vi "IMAQdx_AbsImage_Flea3_v4.5.vi"() -> ()   [LabVIEW 2013] (continued)
+combWidthF/2))\tODTpowHLat(DipPowHLat)\t1\tVimaging\t0\t0\t0\t1\t1\t1\tbMOTdelta(MOTdetuning)\tbMOTpow(0.5)\tProbePow\t0\tXshim\tYshim\tZshimVar\tODTpowZ(DipPowZ)\tVimaging\t0\t0\tHimaging\t0\t0\t0\t0\t0\t0\t0\t0\t0\t0\t0\t0\t0\t0\trMOTdelta(-(rMOTstirDetI +stirWidthF/2))\t0\tODTpowXY(DipPowCr)\tvarWaveP2\t0\t0\trMOTpow3\tODTpowX(DipPowX)\tfreq\tHeatingAmp\t0\tSine\tDetuning\tsingleFreqDet\tDoppCoolDet-DoppCoolSweep\tdopCoolT*1000\tDetuning\tsingleFreqStirDet\tsingleFreqStirDet + 20\tSFcoolT*1000\tBlueBN\tBlueLaserProbeBN\tPixisPos(TOF)\tCycle Wait for Move\tEOMmodFreq\tEOMmodAmp\r\ntransmit img\t\tRamp\t1\t.6\t0\t0\t0\t0\t0\t0\t1\t0\t0\t1\t0\t0\t0\t0\t0\t0\t0\t0\t0\t0\t0\t0\t0\t0\t0\t0\t1\t0\t0\t0\t1\t1\t0\tplus_zman\tminus_zman\tcompensation\trMOTcurrF\trMOTpow3\tcombAmplitude(combWidthF)\trMOTdelta(-(rMOTbroadDetuningF +combWidthF/2))\tODTpowHLat(DipPowHLat)\t1\tVimaging\t0\t0\t0\t1\t1\t1\tbMOTdelta(MOTdetuning)\tbMOTpow(0.5)\tProbePow\t0\tXshim\tYshim\tZshimVar\tODTpowZ(DipPowZ)\tVimaging\t0\t0\tHimaging\t0\t0\t0\t0\t0\t0\t0\t0\t0\t0\t0\t0\t0\t0\trMOTdelta(-(rMOTstirDetI +stirWidthF/2))\t0\tODTpowXY(DipPowCr)\tvarWaveP2\t0\t0\trMOTpow3\tODTpowX(DipPowX)\tfreq\tHeatingAmp\t0\tSine\tDetuning\tsingleFreqDet\tDoppCoolDet-DoppCoolSweep\tdopCoolT*1000\tDetuning\tsingleFreqStirDet\tsingleFreqStirDet + 20\tSFcoolT*1000\tBlueBN\tBlueLaserProbeBN\tPixisPos(TOF)\tCycle Wait for Move\tEOMmodFreq\tEOMmodAmp\r\narm PIXIS\t\tRamp\t0\t.007\t0\t0\t0\t0\t0\t0\t1\t0\t0\t1\t1\t0\t0\t0\t1\t1\t0\t0\t0\t0\t0\t0\t0\t0\t0\t0\t1\t0\t0\t0\t1\t1\t0\tplus_zman\tminus_zman\tcompensation\trMOTcurrF\trMOTpow1\tcombAmplitude(combWidthF)\trMOTdelta(-(rMOTbroadDetuningF +combWidthF/2))\tODTpowHLat(DipPowHLat)\t1\tVimaging\t0\t0\t0\t1\t1\t1\tbMOTdelta(MOTdetuning)\tbMOTpow(0.5)\tProbePow\t0\tXshim\tYshim\tZshimVar\tODTpowZ(DipPowZ)\tVimaging\t0\t0\tHimaging\t0\t0\t0\t0\t0\t0\t0\t0\t0\t0\t0\t0\t0\t0\trMOTdelta(-(rMOTstirDetI +stirWidthF/2))\t0\tODTpowXY(DipPowCr)\tvarWaveP2\t0\t0\trMOTpow1\tODTpowX(DipPowX)\tfreq\tHeatingAmp\t0\tSine\tDetuning\tsingleFreqDet\tDoppCoolDet-DoppCoolSweep\tdopCoolT*1000\tDetuning\tsingleFreqStirDet\tsingleFreqStirDet + 20\tSFcoolT*1000\tBlueBN\tBlueLaserProbeBN\tPixisPos(TOF)\tCycle Wait for Move\tEOMmodFreq\tEOMmodAmp\r\narm FLEA\t\tRamp\t1\t44e-6\t0\t0\t0\t0\t0\t0\t1\t0\t0\t1\t1\t0\t0\t0\t1\t1\t0\t0\t0\t0\t0\t0\t0\t0\t0\t0\t1\t0\t0\t0\t1\t0\t0\tplus_zman\tminus_zman\tcompensation\trMOTcurrF\trMOTpow1\tcombAmplitude(combWidthF)\trMOTdelta(-(rMOTbroadDetuningF +combWidthF/2))\tODTpowHLat(DipPowHLat)\t1\tVimaging\t0\t0\t0\t1\t1\t0\tbMOTdelta(MOTdetuning)\tbMOTpow(0.5)\tProbePow\t0\tXshim\tYshim\tZshimVar\tODTpowZ(DipPowZ)\tVimaging\t0\t0\tHimaging\t0\t0\t0\t0\t0\t0\t0\t0\t0\t0\t0\t0\t0\t0\trMOTdelta(-(rMOTstirDetI +stirWidthF/2))\t0\tODTpowXY(DipPowCr)\tvarWaveP2\t0\t0\trMOTpow1\tODTpowX(DipPowX)\tfreq\tHeatingAmp\t0\tSine\tDetuning\tsingleFreqDet\tDoppCoolDet-DoppCoolSweep\tdopCoolT*1000\tDetuning\tsingleFreqStirDet\tsingleFreqStirDet + 20\tSFcoolT*1000\tBlueBN\tBlueLaserProbeBN\tPixisPos(TOF)\tCycle Wait for Move\tEOMmodFreq\tEOMmodAmp\r\nprobe img\t\tRamp\t1\t10e-6\t0\t0\t0\t0\t0\t0\t1\t0\t1\t1\t1\t0\t0\t1\t1\t1\t0\t0\t0\t0\t0\t0\t0\t0\t0\t0\t1\t0\t0\t0\t1\t0\t0\tplus_zman\tminus_zman\tcompensation\trMOTcurrF\trMOTpow1\tcombAmplitude(combWidthF)\trMOTdelta(-(rMOTbroadDetuningF +combWidthF/2))\tODTpowHLat(DipPowHLat)\t1\tVimaging\t0\t0\t0\t1\t0\t0\tbMOTdelta(MOTdetuning)\tbMOTpow(0.5)\tProbePow\t0\tXshim\tYshim\tZshimVar\tODTpowZ(DipPowZ)\tVimaging\t0\t0\tHimaging\t0\t0\t0\t0\t0\t0\t0\t0\t0\t0\t0\t0\t0\t0\trMOTdelta(-(rMOTstirDetI +stirWidthF/2))\t0\tODTpowXY(DipPowCr)\tvarWaveP2\t0\t0\trMOTpow1\tODTpowX(DipPowX)\tfreq\tHeatingAmp\t0\tSine\tDetuning\tsingleFreqDet\tDoppCoolDet-DoppCoolSweep\tdopCoolT*1000\tDetuning\tsingleFreqStirDet\tsingleFreqStirDet + 20\tSFcoolT*1000\tBlueBN\tBlueLaserProbeBN\tPixisPos(TOF)\tCycle Wait for Move\tEOMmodFreq\tEOMmodAmp\r\nprobe img\t\tRamp\t0\t2.8e-3\t0\t0\t0\t0\t0\t0\t1\t0\t0\t1\t1\t0\t0\t0\t1\t1\t0\t0\t0\t0\t0\t0\t0\t0\t0\t0\t1\t0\t0\t0\t1\t1\t0\tplus_zman\tminus_zman\tcompensation\trMOTcurrF\trMOTpow1\tcombAmplitude(combWidthF)\trMOTdelta(-(rMOTbroadDetuningF +combWidthF/2))\tODTpowHLat(DipPowHLat)\t1\tVimaging\t0\t0\t0\t1\t1\t1\tbMOTdelta(MOTdetuning)\tbMOTpow(0.5)\tProbePow\t0\tXshim\tYshim\tZshimVar\tODTpowZ(DipPowZ)\tVimaging\t0\t0\tHimaging\t0\t0\t0\t0\t0\t0\t0\t0\t0\t0\t0\t0\t0\t0\trMOTdelta(-(rMOTstirDetI +stirWidthF/2))\t0\tODTpowXY(DipPowCr)\tvarWaveP2\t0\t0\trMOTpow1\tODTpowX(DipPowX)\tfreq\tHeatingAmp\t0\tSine\tDetuning\tsingleFreqDet\tDoppCoolDet-DoppCoolSweep\tdopCoolT*1000\tDetuning\tsingleFreqStirDet\tsingleFreqStirDet + 20\tSFcoolT*1000\tBlueBN\tBlueLaserProbeBN\tPixisPos(TOF)\tCycle Wait for Move\tEOMmodFreq\tEOMmodAmp\r\ntransmit img\t\tRamp\t1\t.585\t0\t0\t0\t0\t0\t0\t1\t0\t0\t1\t1\t0\t0\t0\t1\t1\t0\t0\t0\t0\t0\t0\t0\t0\t0\t0\t1\t0\t0\t0\t1\t1\t0\tplus_zman\tminus_zman\tcompensation\trMOTcurrF\trMOTpow1\tcombAmplitude(combWidthF)\trMOTdelta(-(rMOTbroadDetuningF +combWidthF/2))\tODTpowHLat(DipPowHLat)\t1\tVimaging\t0\t0\t0\t1\t1\t1\tbMOTdelta(MOTdetuning)\tbMOTpow(0.5)\tProbePow\t0\tXshim\tYshim\tZshimVar\tODTpowZ(DipPowZ)\tVimaging\t0\t0\tHimaging\t0\t0\t0\t0\t0\t0\t0\t0\t0\t0\t0\t0\t0\t0\trMOTdelta(-(rMOTstirDetI +stirWidthF/2))\t0\tODTpowXY(DipPowCr)\tvarWaveP2\t0\t0\trMOTpow1\tODTpowX(DipPowX)\tfreq\tHeatingAmp\t0\tSine\tDetuning\tsingleFreqDet\tDoppCoolDet-DoppCoolSweep\tdopCoolT*1000\tDetuning\tsingleFreqStirDet\tsingleFreqStirDet + 20\tSFcoolT*1000\tBlueBN\tBlueLaserProbeBN\tPixisPos(TOF)\tCycle Wait for Move\tEOMmodFreq\tEOMmodAmp\r\ntransmit img\t\tRamp\t1\t.015\t0\t0\t0\t0\t0\t0\t1\t0\t0\t1\t1\t0\t0\t0\t1\t1\t0\t0\t0\t0\t0\t0\t0\t0\t0\t0\t1\t0\t0\t0\t1\t1\t0\tplus_zman\tminus_zman\tcompensation\trMOTcurrF\trMOTpow1\tcombAmplitude(combWidthF)\trMOTdelta(-(rMOTbroadDetuningF +combWidthF/2))\tODTpowHLat(DipPowHLat)\t1\tVimaging\t0\t0\t0\t1\t1\t1\tbMOTdelta(MOTdetuning)\tbMOTpow(0.5)\tProbePow\t0\tXshim\tYshim\tZshimVar\tODTpowZ(DipPowZ)\tVimaging\t0\t0\tHimaging\t0\t0\t0\t0\t0\t0\t0\t0\t0\t0\t0\t0\t0\t0\trMOTdelta(-(rMOTstirDetI +stirWidthF/2))\t0\tODTpowXY(DipPowCr)\tvarWaveP2\t0\t0\trMOTpow1\tODTpowX(DipPowX)\tfreq\tHeatingAmp\t0\tSine\tDetuning\tsingleFreqDet\tDoppCoolDet-DoppCoolSweep\tdopCoolT*1000\tDetuning\tsingleFreqStirDet\tsingleFreqStirDet + 20\tSFcoolT*1000\tBlueBN\tBlueLaserProbeBN\tPixisPos(TOF)\tCycle Wait for Move\tEOMmodFreq\tEOMmodAmp\r\narm PIXIS\t\tRamp\t0\t.007\t0\t0\t0\t0\t0\t0\t1\t0\t0\t1\t1\t0\t0\t0\t1\t1\t0\t0\t0\t0\t0\t0\t0\t0\t0\t0\t1\t0\t0\t0\t1\t0\t0\tplus_zman\tminus_zman\tcompensation\trMOTcurrF\trMOTpow1\tcombAmplitude(combWidthF)\trMOTdelta(-(rMOTbroadDetuningF +combWidthF/2))\tODTpowHLat(DipPowHLat)\t1\tVimaging\t0\t0\t0\t1\t1\t1\tbMOTdelta(MOTdetuning)\tbMOTpow(0.5)\tProbePow\t0\tXshim\tYshim\tZshimVar\tODTpowZ(DipPowZ)\tVimaging\t0\t0\tHimaging\t0\t0\t0\t0\t0\t0\t0\t0\t0\t0\t0\t0\t0\t0\trMOTdelta(-(rMOTstirDetI +stirWidthF/2))\t0\tODTpowXY(DipPowCr)\tvarWaveP2\t0\t0\trMOTpow1\tODTpowX(DipPowX)\tfreq\tHeatingAmp\t0\tSine\tDetuning\tsingleFreqDet\tDoppCoolDet-DoppCoolSweep\tdopCoolT*1000\tDetuning\tsingleFreqStirDet\tsingleFreqStirDet + 20\tSFcoolT*1000\tBlueBN\tBlueLaserProbeBN\tPixisPos(TOF)\tCycle Wait for Move\tEOMmodFreq\tEOMmodAmp\r\narm FLEA\t\tRamp\t1\t44e-6\t0\t0\t0\t0\t0\t0\t1\t0\t0\t1\t1\t0\t0\t0\t1\t1\t0\t0\t0\t0\t0\t0\t0\t0\t0\t0\t1\t0\t0\t0\t1\t0\t0\tplus_zman\tminus_zman\tcompensation\trMOTcurrF\trMOTpow1\tcombAmplitude(combWidthF)\trMOTdelta(-(rMOTbroadDetuningF +combWidthF/2))\tODTpowHLat(DipPowHLat)\t1\tVimaging\t0\t0\t0\t1\t1\t0\tbMOTdelta(MOTdetuning)\tbMOTpow(0.5)\tProbePow\t0\tXshim\tYshim\tZshimVar\tODTpowZ(DipPowZ)\tVimaging\t0\t0\tHimaging\t0\t0\t0\t0\t0\t0\t0\t0\t0\t0\t0\t0\t0\t0\trMOTdelta(-(rMOTstirDetI +stirWidthF/2))\t0\tODTpowXY(DipPowCr)\tvarWaveP2\t0\t0\trMOTpow1\tODTpowX(DipPowX)\tfreq\tHeatingAmp\t0\tSine\tDetuning\tsingleFreqDet\tDoppCoolDet-DoppCoolSweep\tdopCoolT*1000\tDetuning\tsingleFreqStirDet\tsingleFreqStirDet + 20\tSFcoolT*1000\tBlueBN\tBlueLaserProbeBN\tPixisPos(TOF)\tCycle Wait for Move\tEOMmodFreq\tEOMmodAmp\r\nbg img\t\tRamp\t1\t10e-6\t0\t0\t0\t0\t0\t0\t1\t0\t0\t1\t1\t0\t0\t0\t1\t1\t0\t0\t0\t0\t0\t0\t0\t0\t0\t0\t1\t0\t0\t0\t1\t0\t0\tplus_zman\tminus_zman\tcompensation\trMOTcurrF\trMOTpow1\tcombAmplitude(combWidthF)\trMOTdelta(-(rMOTbroadDetuningF +combWidthF/2))\tODTpowHLat(DipPowHLat)\t1\tVimaging\t0\t0\t0\t1\t0\t0\tbMOTdelta(MOTdetuning)\tbMOTpow(0.5)\tProbePow\t0\tXshim\tYshim\tZshimVar\tODTpowZ(DipPowZ)\tVimaging\t0\t0\tHimaging\t0\t0\t0\t0\t0\t0\t0\t0\t0\t0\t0\t0\t0\t0\trMOTdelta(-(rMOTstirDetI +stirWidthF/2))\t0\tODTpowXY(DipPowCr)\tvarWaveP2\t0\t0\trMOTpow1\tODTpowX(DipPowX)\tfreq\tHeatingAmp\t0\tSine\tDetuning\tsingleFreqDet\tDoppCoolDet-DoppCoolSweep\tdopCoolT*1000\tDetuning\tsingleFreqStirDet\tsingleFreqStirDet + 20\tSFcoolT*1000\tBlueBN\tBlueLaserProbeBN\tPixisPos(TOF)\tCycle Wait for Move\tEOMmodFreq\tEOMmodAmp\r\nbg img\t\tRamp\t0\t1e-4\t0\t0\t0\t0\t0\t0\t1\t0\t0\t1\t1\t0\t0\t0\t1\t1\t0\t0\t0\t0\t0\t0\t0\t0\t0\t0\t1\t0\t0\t0\t1\t1\t0\tplus_zman\tminus_zman\tcompensation\trMOTcurrF\trMOTpow1\tcombAmplitude(combWidthF)\trMOTdelta(-(rMOTbroadDetuningF +combWidthF/2))\tODTpowHLat(DipPowHLat)\t1\tVimaging\t0\t0\t0\t1\t1\t1\tbMOTdelta(MOTdetuning)\tbMOTpow(0.5)\tProbePow\t0\tXshim\tYshim\tZshimVar\tODTpowZ(DipPowZ)\tVimaging\t0\t0\tHimaging\t0\t0\t0\t0\t0\t0\t0\t0\t0\t0\t0\t0\t0\t0\trMOTdelta(-(rMOTstirDetI +stirWidthF/2))\t0\tODTpowXY(DipPowCr)\tvarWaveP2\t0\t0\trMOTpow1\tODTpowX(DipPowX)\tfreq\tHeatingAmp\t0\tSine\tDetuning\tsingleFreqDet\tDoppCoolDet-DoppCoolSweep\tdopCoolT*1000\tDetuning\tsingleFreqStirDet\tsingleFreqStirDet + 20\tSFcoolT*1000\tBlueBN\tBlueLaserProbeBN\tPixisPos(TOF)\tCycle Wait for Move\tEOMmodFreq\tEOMmodAmp\r\ntransmit img\t\tRamp\t1\t.6\t0\t0\t0\t0\t0\t0\t1\t0\t0\t1\t1\t0\t0\t0\t1\t1\t0\t0\t0\t0\t0\t0\t0\t0\t0\t0\t1\t0\t0\t0\t1\t1\t0\tplus_zman\tminus_zman\tcompensation\trMOTcurrF\trMOTpow1\tcombAmplitude(combWidthF)\trMOTdelta(-(rMOTbroadDetuningF +combWidthF/2))\tODTpowHLat(DipPowHLat)\t1\tVimaging\t0\t0\t0\t1\t1\t1\tbMOTdelta(MOTdetuning)\tbMOTpow(0.5)\tProbePow\t0\tXshim\tYshim\tZshimVar\tODTpowZ(DipPowZ)\tVimaging\t0\t0\tHimaging\t0\t0\t0\t0\t0\t0\t0\t0\t0\t0\t0\t0\t0\t0\trMOTdelta(-(rMOTstirDetI +stirWidthF/2))\t0\tODTpowXY(DipPowCr)\tvarWaveP2\t0\t0\trMOTpow1\tODTpowX(DipPowX)\tfreq\tHeatingAmp\t0\tSine\tDetuning\tsingleFreqDet\tDoppCoolDet-DoppCoolSweep\tdopCoolT*1000\tDetuning\tsingleFreqStirDet\tsingleFreqStirDet + 20\tSFcoolT*1000\tBlueBN\tBlueLaserProbeBN\tPixisPos(TOF)\tCycle Wait for Move\tEOMmodFreq\tEOMmodAmp\r\nalignment\t\tRamp\t1\t.1\t1\t1\t1\t1\t1\t1\t1\t0\t1\t0\t1\t0\t1\t1\t1\t1\t0\t0\t0\t0\t0\t0\t0\t0\t1m\t0\t1\t0\t1\t0\t0\t1\t1\tplus_zman\tminus_zman\tcompensation\tMOTcurrent\trMOTpow1\tcombAmplitude(combWidthI)\trMOTdelta(-(rMOTbroadDetuningI +combWidthI/2))\tODTpowHLat(DipPowHLat)\t1\t0\t1\t1\t0\t1\t1\t1\tbMOTdelta(MOTdetuning)\tbMOTpow(MOTPow)\tProbePow\t0\tXshim\tYshim\tZshim\tODTpowZ(DipPowZ2)\t0\t1\t0\t0\t1\t1\t0\t0\t0\t0\t0\t0\t0\t0\t0\t0\t0\t0\trMOTdelta(-(rMOTstirDetI +stirWidthI/2))\t0\tODTpowXY(DipPowCr)\tvarWaveP2\t0\t0\trMOTpow3\tODTpowX(DipPowX)\tfreq\tHeatingAmp\t0\tSine\tRamp\tsingleFreqDet\tsingleFreqDetF\tSFcoolT*1000\tRamp\tsingleFreqStirDet\tsingleFreqStirDetF\tSFcoolT*1000\tBlueBN\tBlueLaserBeatnote\tPixisPos(TOF)\tCycle Wait for Move\tEOMmodFreq\tEOMmodAmp\r\n\r\n\r\n"
  in  "Flea Wave Name":string="Test_Img"
  in  "Save files to archive?":bool
  out "Timeout":bool=TRUE
  out "Trigger Overrun":bool=TRUE
  in  "Source of File Data":refnum<k21>="\\\\192.168.137.181\\VariableLibrary\\Instruction String"
  in  "Timeout (ms)":u32=20000
  in  "Gain":dbl
  in  "Shutter speed":dbl=0.03
  in  "PIXIS Magnification":dbl=5.48
  in  "PIXIS Image direction":enum16{"XY", "XZ"}(ring)
  in  "PIXIS Imaging technique":enum16{"Absorption", "Fluorescence", "RawImage"}(ring)
  in  "SPE File Path":path=path "C:/Users/Lab/Documents/LightField/LabviewTemp.spe"
  in  "Send PIXIS data to Igor?":bool
  in  "PIXIS File Parameters":T1={"Data Root"=path "I:/Data", "Index"=4, "Instrument"="PIXIS"} {"Index" format="%04d"}
  in  "Source of Wavemeter Data":refnum<k21>="\\\\WS7PC\\VariableLibrary\\Frequency"
  in  "Accept wavelength from remote system":bool=TRUE
  in  "Flea Raw image to view":u16(ring) items=["Clear", "Absorbtion", "Probe", "Background"]
  in  "Update Graphics":bool=TRUE
  out "Flea Raw Image":u16[][](graph)
  out "Flea Processed Image":sgl[][](graph)
  out "PIXIS Processed Image":sgl[][](graph)
  out "PIXIS Raw Image":u16[][](graph)
  in  "PIXIS Raw image to view":u16(ring)=1 items=["Clear", "Absorbtion", "Probe", "Background"]
  out "Camera Error":errorcluster={"status"=FALSE, "code"=-1074360293, "source"="IMAQdx Get Image2.vi"}
  out "DDE Error":errorcluster={"status"=TRUE, "code"=14012, "source"="DDE Execute: DMLERR_NOTPROCESSED"}
  out "Status Array":T4(array[cluster])=[{"AcquisitionInProgress"=FALSE, "BufferCount"=0, "LastBufferNumber"=4294967292, "LostBufferCount"=0}, {"AcquisitionInProgress"=TRUE, "BufferCount"=0, "LastBufferNumber"=4294967292, "LostBufferCount"=0}, {"AcquisitionInProgress"=TRUE, "BufferCount"=1, "LastBufferNumber"=0, "LostBufferCount"=0}, {"AcquisitionInProgress"=TRUE, "BufferCount"=2, "LastBufferNumber"=1, "LostBufferCount"=0}, {"AcquisitionInProgress"=TRUE, "BufferCount"=3, "LastBufferNumber"=2, "LostBufferCount"=0}, {"AcquisitionInProgress"=TRUE, "BufferCount"=4, "LastBufferNumber"=3, "LostBufferCount"=0}]
  in  "SPE Load Error In":errorcluster
  out "DataBlock Info":T5={"frame count"=4, "frame size"=524288, "frame stride"=524288, "N ROI"=1, "ROI widths"=[512], "ROI heights"=[512], "ROI sizes"=[524288], "ROI strides"=[524288]}
  out "DS Error":errorcluster
  out "XML Parse Errors":string
  out "Data Array Size":i32=1
  out "SPE Load Error Out":errorcluster
  out "Flea Path":path=path "I:/Data/Flea3_20S4Mtemp.ibw"
  out "PIXIS Path":path=path "C:/Experiment/Data/PIXIStemp.ibw"
  out "PIXIS Images":u16[][][](array[numeric])
  out "Flea Images":u16[][][](array[numeric])
  out "Buffer Number":u32=4294967294
  out "Flea Frames":i32
  out "Flea Loop":i32=1
  # "Image Acquisition v4.5"
  # "Experimental Parameters"
  # "These are only get set on 1st run.\nUse a Gain of 0, Shutter Speed not used"
  # "In both techniques 3 images\nare aquired, but in Fluorescense\nthe 3rd is discarded"
  # "Sr: .663  is XZ a\n     .898 is XZ b\n      5.48 is XY"
  # "Obsolete: (now done with network variables)\nWhen paramaters are accepted from a remote system a DataSockets server\nmust be running on this machine (in start menu in National Instruments folder)"
  # "Camera configuration"
  # "File configuration"
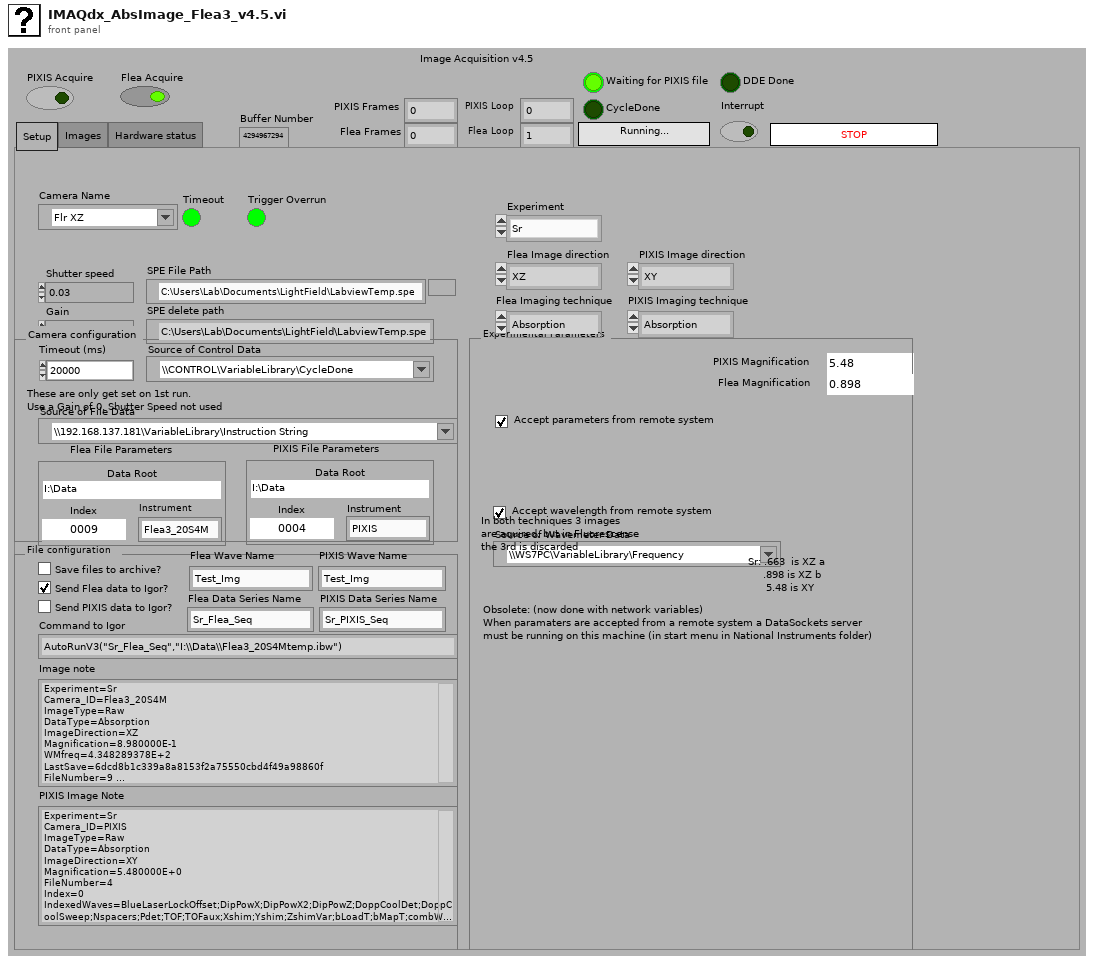
[diagram p1: front panel]
types:
  T1 = typedef "FileName_Cluster.ctl" = cluster{"Data Root":path, "Index":u32, "Instrument":string}
  T2 = typedef "IMAQdx.ctl" = refnum<k21>
  T3 = enum16{"Rubidium I", "Rubidium II", "RbLi", "RbYb", "Sr"}
  T4 = cluster{"AcquisitionInProgress":bool, "BufferCount":u32, "LastBufferNumber":u32, "LostBufferCount":u32}[]
  T5 = cluster{"frame count":i64, "frame size":i64, "frame stride":i64, "N ROI":i64, "ROI widths":i64[], "ROI heights":i64[], "ROI sizes":i64[], "ROI strides":i64[]}
  T6 = typedef "NI_Vision_Acquisition_Software.lvlib/IMAQdx Acquisition Mode.ctl" = enum32{"One Shot", "Continuous"}
  T7 = typedef "Image Type" = u32
  T8 = typedef "IMAQ Image.ctl" = refnum<image>
  T9 = cluster{"AcquisitionInProgress":bool, "BufferCount":u32, "LastBufferNumber":u32, "LostBufferCount":u32}
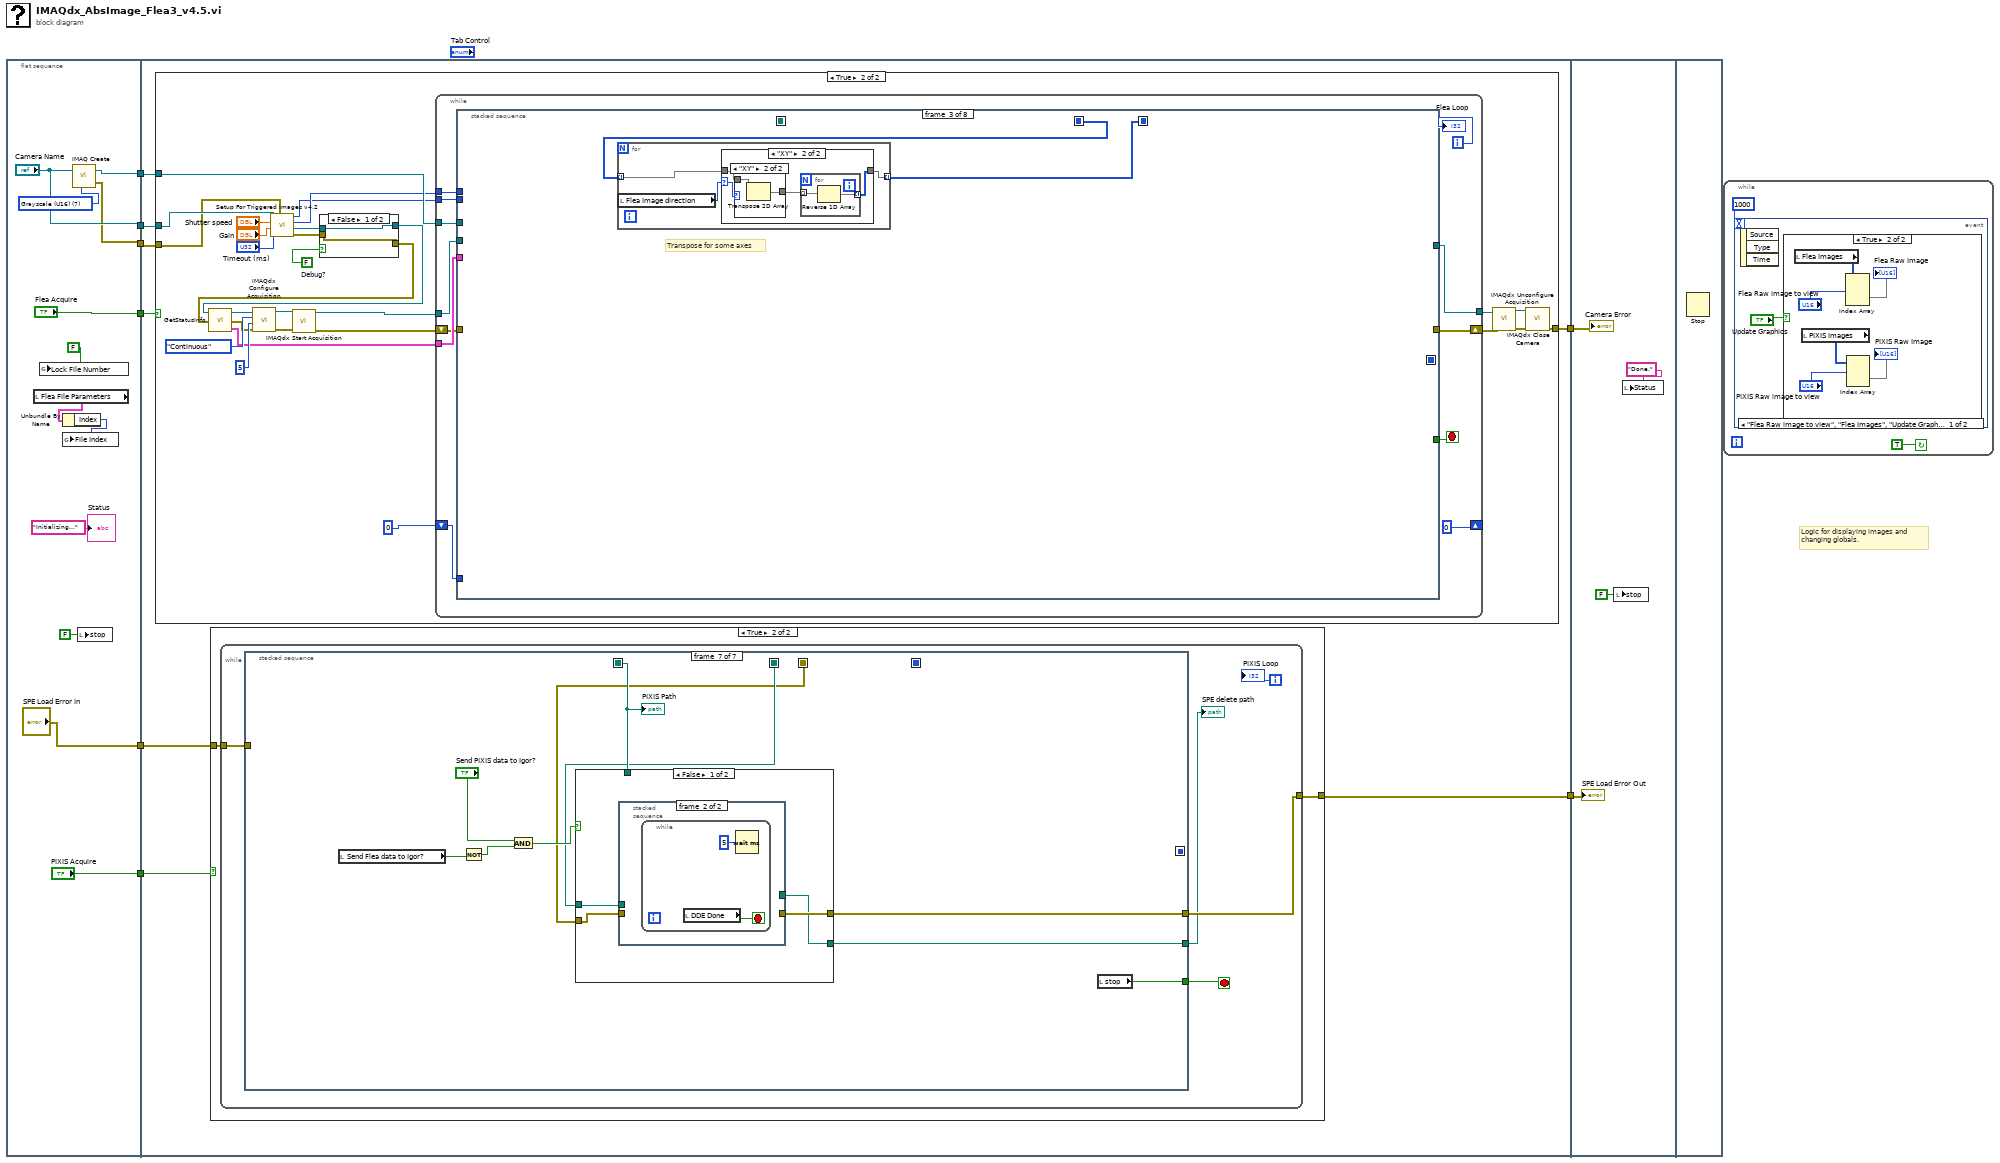
[diagram p0: block diagram]
diagram:
  # "Logic for displaying images and\nchanging globals."
  n1 = flat-sequence {
    tunnel: [w16] -> w8
    tunnel: ["Camera Name"] -> w7
    tunnel: [w14] -> w6
    tunnel: ["SPE Load Error In"] -> w5
    tunnel: ["PIXIS Acquire"] -> w3
    tunnel: ["Flea Acquire"] -> w1
    tunnel: w7 -> [w28]
    tunnel: w8 -> [w26]
    tunnel: w6 -> [w27]
    tunnel: w5 -> [w25]
    tunnel: [w24] -> w4
    tunnel: w3 -> [w23]
    tunnel: [w22] -> w2
    tunnel: w1 -> [w21]
    tunnel: w4 -> [w463]
    tunnel: w2 -> [w462]
    frame #0 {
      w13 = T7 7 items=["Grayscale (U8)", "Grayscale (I16)", "Grayscale (SGL)", "Complex (CSG)", "RGB (U32)", "HSL (U32)", "RGB (U64)", "Grayscale (U16)"] ("Image Type")
      n2 = local read "Flea File Parameters"() -> (w17:T1)
      n3 = global write "FileInfo_Global.vi" "Lock File Number"(FALSE) -> ()
      n4 = Unbundle By Name(w17) -> ("Index"=w18:u32)
      n5 = global write "FileInfo_Global.vi" "File Index"(w18) -> ()
      n6 = call "IMAQ Create"("Image Name"="Camera Name", "Image Type"=w13) -> ("New Image"=w16:T8, "error out"=w14:errorcluster)  [unwired: 2 in, 1 out]
      n7 = local write "stop"(FALSE ("stop")) -> ()
      "Status" <- "Initializing..."
    }
    frame #1 {
      n8 = case shown="True" w21 {
        tunnel: w28 -> [_ w43]
        tunnel: w27 -> [w29 w42]
        tunnel: w26 -> [_ w40]
        tunnel: [w29 w32] -> w22
        frame False {
        }
        frame True {
          w50 = FALSE  # Debug?
          n9 = call "Setup For Triggered Images v4.2.vi"("error in"=w42, "Timeout (ms)"="Timeout (ms)", "Gain"="Gain", "Shutter speed"="Shutter speed", "Camera Name"=w43) -> ("Error out"=w51:errorcluster, "Session Out"=w52:T2, "Height"=w39:u32, "Width"=w38:u32)
          n10 = case shown="False" w50 {
            tunnel: [w58 w63] -> w49
            tunnel: [w59 w62] -> w46
            tunnel: w52 -> [w58 w61]
            tunnel: w51 -> [w59 w60]
            frame False {
            }
            frame True {
              n11 = call "CheckCameraAttributes-CDH.vi"("error in"=w60, "Camera Name"=w61) -> ("error out"=w62:errorcluster, "Session Out"=w63:T2)
            }
          }
          n12 = call "GetStatusInfo.vi"("error in"=w46, "Camera In"=w49) -> ("Status Info"=w37:T9, "error out"=w47:errorcluster, "Camera Out"=w48:T2)  [unwired: 1 in]
          n13 = call <vilib>:"IMAQdx Configure Acquisition.vi"("error in"=w47, "Number of Buffers"=u32 5, "Continuous?"=IMAQdx_Acquisition_Mode."Continuous", "Session In"=w48) -> ("error out"=w44:errorcluster, "Session Out"=w45:T2)  [unwired: 6 in]
          n14 = call <vilib>:"IMAQdx Start Acquisition.vi"("error in"=w44, "Session In"=w45) -> ("error out"=w35:errorcluster, "Session Out"=w41:T2)  [unwired: 8 out]
          n15 = while {
            tunnel: w41 -> [w73]
            tunnel: w40 -> [w72]
            tunnel: w39 -> [w71]
            tunnel: w38 -> [w70]
            tunnel: w37 -> [w69]
            tunnel: [w68] -> w31
            shift-right: [0] -> _
            shift-left: 0 -> [w67]
            shift-right: [w64] -> w34
            shift-left: w35 -> [w65]
            i -> [w75]
            stop <- w74 stop-if-true
            n16 = stacked-sequence {
              seq-local: [_ _ _ w178 _ _ _ _] -> [_ _ _ _ _ w248 _ _]
              seq-local: [_ _ _ _ _ w244 _ _] -> [_ _ _ _ _ _ _ w258]
              seq-local: [_ w81 _ _ _ _ _ _] -> [_ _ w152 _ _ _ _ _]
              seq-local: [_ _ w151 _ _ _ _ _] -> [_ _ _ w169 _ _ _ _]
              tunnel: [_ _ _ _ _ _ _ "stop"] -> w74
              tunnel: w73 -> [_ w93 _ _ _ _ _ _]
              tunnel: w72 -> [_ w92 _ _ _ _ _ _]
              tunnel: w71 -> [_ w91 _ _ _ _ _ _]
              tunnel: w70 -> [_ w90 _ _ _ _ _ _]
              tunnel: w69 -> [_ w88 _ _ _ _ _ _]
              tunnel: [_ w87 _ _ _ _ _ _] -> w68
              tunnel: [_ w84 _ _ _ _ _ _] -> w64
              tunnel: w67 -> [_ w86 _ _ _ _ _ _]
              tunnel: w65 -> [_ w85 _ _ _ _ _ _]
              frame #0 {
                n17 = local read "Send Flea data to Igor?"() -> (w76:bool)
                n18 = local write "Flea Frames"(0) -> ()
                n19 = local write "Status"("Running...") -> ()
                n20 = case shown="True" w76 {
                  frame False {
                    n21 = local write "DDE Done"(TRUE ("DDE Done")) -> ()
                  }
                  frame True {
                    "DDE Done" <- FALSE
                  }
                }
              }
              frame #1 {
                n22 = Build Array(w88) -> (w89:T4)
                n23 = Initialize Array(u16 0, 4, w91, w90) -> (w95:u16[][][])
                n24 = while {
                  shift-right: [w105] -> _
                  shift-left: _ -> [w129]
                  tunnel: [w113] -> w87
                  tunnel: [w110] -> w83
                  shift-right: [w120] -> _
                  shift-left: w86 -> [w107]
                  shift-right: [w125] -> w81
                  shift-left: w95 -> [w126]
                  shift-right: [w108] -> w94
                  shift-left: w89 -> [w109]
                  tunnel: w93 -> [w104]
                  tunnel: w92 -> [w103]
                  tunnel: w85 -> [w102]
                  stop <- w116 continue-if-true
                  # "(Timeout code = -1074364414, IMAQ)\n(Timeout code = -1074360293, IMAQdx)\nDon't timeout waiting for first\nimage."
                  n25 = call <vilib>:"IMAQdx Grab.vi"("error in"=w102, "Wait for Next Buffer? (Yes)"=TRUE, "Image In"=w103, "Session In"=w104) -> ("error out"=w124:errorcluster, "Buffer Number Out"=w105:u32, "Image Out"=w119:T8, "Session Out"=w112:T2)  [unwired: 4 out]
                  "Buffer Number" <- w105
                  n26 = Unbundle By Name(w124) -> ("code"=w133:i32)
                  n27 = call "IMAQ ImageToArray"("Image"=w119) -> ("Image Pixels (U16)"=w118:u16[][])  [unwired: 2 in, 5 out]
                  n28 = case shown="-1074364414, -1074360293" w133 {
                    tunnel: w124 -> [w138 w142]
                    tunnel: [w138 w141] -> w111
                    tunnel: [FALSE TRUE] -> w134
                    tunnel: w107 -> [w136 w140]
                    tunnel: [w135 w139] -> w120
                    frame 0, Default {
                      n29 = Increment(x=w136) -> (x+1=w135:i32)
                    }
                    frame -1074364414, -1074360293 {
                      n30 = case shown="1, Default" w140 {
                        tunnel: [w144 w150] -> w141
                        tunnel: w142 -> [w146 w150]
                        tunnel: w140 -> [w145 w149]
                        tunnel: [w145 w148] -> w139
                        frame 0 {
                          n31 = Bundle By Name(cluster=w146, "status"=FALSE) -> (w144:errorcluster)
                        }
                        frame 1, Default {
                          n32 = Increment(x=w149) -> (x+1=w148:i32)
                        }
                      }
                    }
                  }
                  "Timeout" <- w134
                  n33 = Subtract(x=w105, y=w129) -> (x-y=w130:u32)
                  n34 = Not Equal?(x=u32 1, y=w130) -> (x != y?=→"Trigger Overrun":bool)
                  n35 = Replace Array Subset(array=w126, new element=w118, index (dim 0)=w107) -> (w125:u16[][][])  [unwired: 2 in]
                  n36 = Unbundle By Name(w111) -> ("status"=w128:bool)
                  n37 = Greater?(x=4, y=w120) -> (0:w121:bool)
                  n38 = Not(x=w128) -> (.not. x?=w127:bool)
                  n39 = call "GetStatusInfo.vi"("error in"=w111, "Camera In"=w112) -> ("Status Info"=w106:T9, "error out"=w110:errorcluster, "Camera Out"=w113:T2)  [unwired: 1 in]
                  n40 = And(x=w127, y=w121) -> (x .and. y?=w117:bool)
                  n41 = Not(x="Interrupt") -> (.not. x?=w114:bool)
                  n42 = Insert Into Array(array=w109, new element=w106) -> (w108:T4)  [unwired: 1 in]
                  n43 = local write "Camera Error"(w110) -> ()
                  n44 = And(x=w117, y=w114) -> (x .and. y?=w116:bool)
                  "Flea Frames" <- w107
                }
                "Flea Images" <- w81
                "Status Array" <- w94
                n45 = Unbundle By Name(w83) -> ("code"=w82:i32)
                n46 = case shown="-1074364414, -1074360293" w82 {
                  tunnel: [w98 w100] -> w84
                  tunnel: w83 -> [w98 w99]
                  frame 0, Default {
                  }
                  frame -1074364414, -1074360293 {
                    n47 = Bundle By Name(cluster=w99, "status"=FALSE) -> (w100:errorcluster)
                  }
                }
              }
              frame #2 {
                # "Transpose for some axes"
                n48 = for {
                  tunnel: w152 -> [w154] mode=indexing
                  tunnel: [w153] -> w151 mode=indexing
                  n49 = local read "Flea Image direction"() -> (w155:enum16{"XY", "XZ"})
                  n50 = case shown="\"XY\"" w155 {
                    selector: w155 -> [_ w157]
                    tunnel: w154 -> [w156 w159]
                    tunnel: [w156 w160] -> w153
                    frame Default {
                    }
                    frame "XY" {
                      n51 = case shown="\"XY\"" w157 {
                        tunnel: w159 -> [w161 w163]
                        tunnel: [w161 w162] -> w158
                        frame Default {
                        }
                        frame "XY" {
                          n52 = Transpose 2D Array(2D array=w163) -> (transposed array=w162:u16[][])
                        }
                      }
                      n53 = for {
                        tunnel: w158 -> [w165] mode=indexing
                        tunnel: [w164] -> w160 mode=indexing
                        n54 = Reverse 1D Array(array=w165) -> (reversed array=w164:u16[])
                      }
                    }
                  }
                }
              }
              frame #3 {
                # "Send to igor a single frame with three images"
                # "For Display only"
                n55 = Array Subset(array=w169, index (dim 0)=1 ("index"), length (dim 0)=3 ("length")) -> (w166:u16[][][])  [unwired: 4 in]
                n56 = Array Size(array=w166) -> (size(s)=w174:i32[])
                n57 = To Single Precision Float(number=w166) -> (single precision float=w175:sgl[][][])
                n58 = case shown="\"Absorption\", Default" "Flea Imaging technique" {
                  tunnel: [w187 w193] -> w179
                  tunnel: w175 -> [w186 w194]